vi "Test Noise Synthesis.vi"() -> ()   [LabVIEW 2015]
uses:
  Controls/Waveforms/Noise/Noise.xctl
  Classes/Waveforms/Noise/Noise.lvclass
  Controls/Filter/Filter.xctl
  Classes/Filter/Filter.lvclass
  Classes/Waveforms/Noise/Noise.lvclass/Noise.ctl
  Classes/Level/Level.lvclass/Level.ctl
  Classes/Waveforms/Noise/Write Freq (Hz).vi
  Classes/Waveforms/Noise/Write Threshold (dB).vi
  Classes/Waveforms/Noise/Read ref (dB).vi
  <vilib>/Utility/file.llb/Read Delimited Spreadsheet (DBL).vi
  Utility VIs/Math VIs/FFT x(t) to dB,Degrees (1D).vi
  Classes/Level/Level.lvclass
panel:
  out "Lfc (dB)":dbl=97.05707780819108
  out "Magnitude 2":T1(graph)
  out "error out":errorcluster
  out "Lmax (dB)":dbl=97.03654195007562
  in  "Fs (Hz)":dbl=50000.0
  out "Magnitude":T2(graph)
  out "Waveform":cluster{"Array":dbl[], "Array":dbl[]}(graph)
  in  "Filter":refnum<class "Filter.lvclass">(xcontrol)=refnum
  in  "Audiogram":path=path "D:/Experiment VIs/Signal Synthesis VIs/4th Generation/Test VIs/test audiogram.tsv"
  in  "Calibration":path=path "C:/Data/Calibrations/TDH-39Left.dBSPL.calib"
  in  "Noise":refnum<class "Noise.lvclass">(xcontrol)=refnum
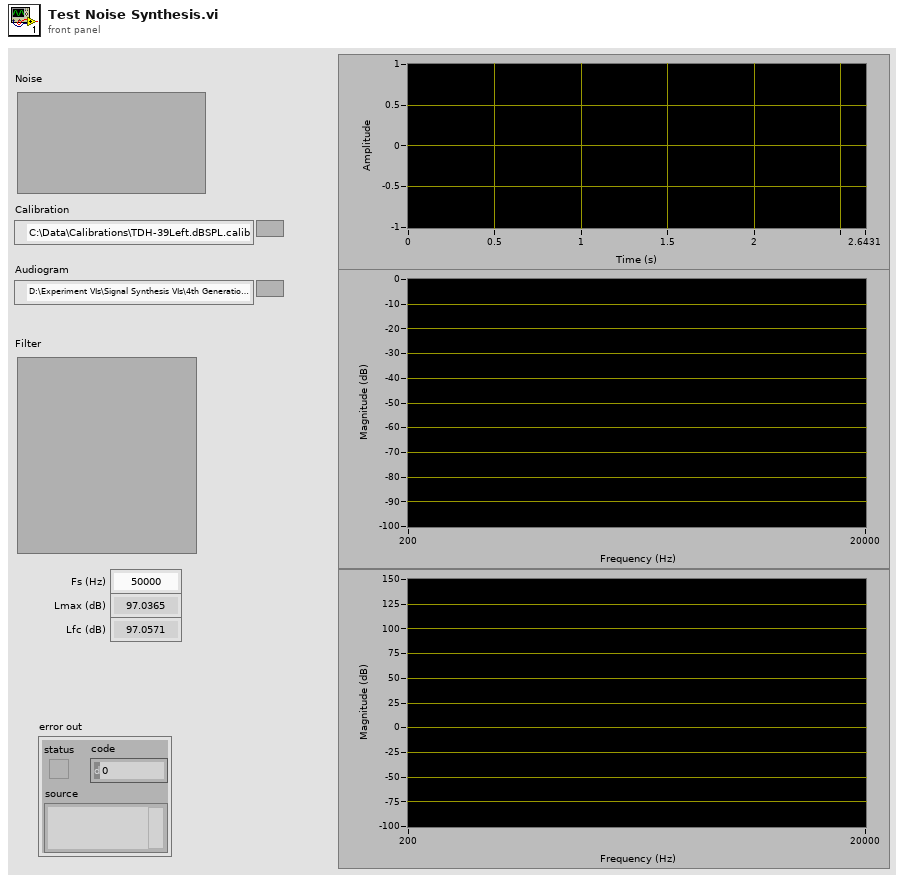
[diagram p1: front panel]
types:
  T1 = cluster{"Freq (Hz)":dbl[], "Magnitude (dB)":dbl[]}[]
  T2 = cluster{"Freq (Hz)":dbl[], "+Freq. Mag of FFT (dB rms)":dbl[]}
  T3 = enum16{"Clear", "Set data", "Reset index", "Get data"}
  T4 = cluster{"Freq (Hz)":dbl[], "Mag (dB SPL)":dbl[], "Phase (deg)":dbl[]}
  T5 = cluster{"Freq (Hz)":dbl[], "Magnitude (dB)":dbl[]}
  T6 = cluster{"Freq (Hz)":dbl[], "Mag (dB SPL)":dbl[]}[]
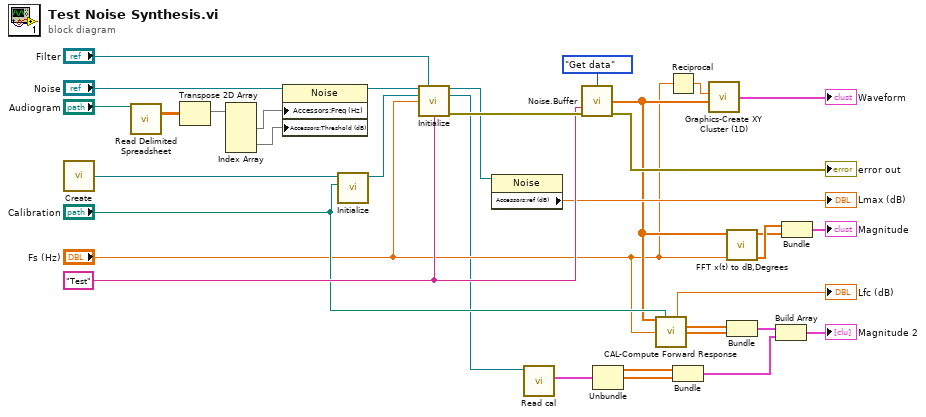
[diagram p0: block diagram]
diagram:
  w27 = "Test" ("Channel Name")
  n1 = call "Create.vi"() -> ("Level"=w34:refnum<class "Level.lvclass">)  [unwired: 15 in]
  n2 = call-poly <vilib>:"Read Delimited Spreadsheet.vi"("file path (dialog if empty)"="Audiogram") -> ("all rows"=w4:dbl[][])  [unwired: 9 in, 5 out]
  n3 = Transpose 2D Array(2D array=w4) -> (transposed array=w3:dbl[][])
  n4 = Index Array(array=w3) -> (element #1=w2:dbl[], element #2=w1:dbl[])  [unwired: 4 in]
  n5 = property class="Noise"(reference="Noise", "Accessors:Freq (Hz)"=w2, "Accessors:Threshold (dB)"=w1) -> (reference out=w6:refnum<class "Noise.lvclass">)  [unwired: 1 in, 1 out]
  n6 = call "Initialize.vi"("Cal file"="Calibration", "Level in"=w34) -> ("Level out"=w31:refnum<class "Level.lvclass">)  [unwired: 8 in, 1 out]
  n7 = call-dynamic "Initialize.vi"("Noise in"=w6, "Filter in"="Filter", "Level in"=w31, "Fs (Hz)"="Fs (Hz)", "Channel Name"=w27) -> ("Noise out"=w21:refnum<class "Noise.lvclass">, "Level out"=w12:refnum<class "Level.lvclass">, "error out"=w28:errorcluster)  [unwired: 7 in, 1 out]
  n8 = property class="Noise"(reference=w21) -> ("Accessors:ref (dB)"=→"Lmax (dB)":dbl)  [unwired: 1 in, 2 out]
  n9 = call "Read cal.vi"("Level in"=w12) -> ("cal"=w11:T4)  [unwired: 8 in, 2 out]
  n10 = call "Noise.Buffer.vi"("Action"=T3."Get data", "Name"=w27, "error in (no error)"=w28) -> ("Data Out"=w18:dbl[], "error out"=→"error out":errorcluster)  [unwired: 11 in]
  n11 = Unbundle(w11) -> ("Freq (Hz)"=w10:dbl[], "Mag (dB SPL)"=w9:dbl[])  [unwired: 1 out]
  n12 = call "CAL-Compute Forward Response.vi"("Y"=w18, "Calibration file"="Calibration", "Fs (Hz)"="Fs (Hz)") -> ("dB SPL"=→"Lfc (dB)":dbl, "Freq (Hz)"=w16:dbl[], "Magnitude (dB)"=w15:dbl[])  [unwired: 8 in, 2 out]
  n13 = Reciprocal(x="Fs (Hz)") -> (1/x=w22:dbl)
  n14 = Bundle("Freq (Hz)"=w10, "Mag (dB SPL)"=w9) -> (w8:cluster{"Freq (Hz)":dbl[], "Mag (dB SPL)":dbl[]})  [unwired: 1 in]
  n15 = call "Graphics-Create XY Cluster (1D).vi"("Array"=w18, "dx"=w22) -> ("XY cluster"=→"Waveform":cluster{"Array":dbl[], "Array":dbl[]})  [unwired: 2 in]
  n16 = call-poly "FFT x(t) to dB,Degrees.vi"("Fs (Hz)"="Fs (Hz)", "X"=w18) -> ("Freq (Hz)"=w25:dbl[], "+Freq. Mag of FFT (dB rms)"=w24:dbl[])  [unwired: 7 in, 1 out]
  n17 = Bundle("Freq (Hz)"=w16, "Magnitude (dB)"=w15) -> (w14:T5)  [unwired: 1 in]
  n18 = Build Array(w14, w8) -> (→"Magnitude 2":T6)
  n19 = Bundle("Freq (Hz)"=w25, "+Freq. Mag of FFT (dB rms)"=w24) -> (→"Magnitude":T2)  [unwired: 1 in]
